vi "SaccadeAnalyser - Main.vi"(8 "error in (no error)":errorcluster, 11 "Data IN":T3={"Impulse Positions"=[{"Start"=5471, "End"=5813, "Impulse Plane"=enum."Yaw", "Impulse Direction +ve?"=FALSE, "Time offset"=0, "Amplitude offset"=0.0}, {"Start"=6974, "End"=7325, "Impulse Plane"=enum."Yaw", "Impulse Direction +ve?"=TRUE, "Time offset"=0, "Amplitude offset"=0.0}, {"Start"=7641, "End"=7980, "Impulse Plane"=enum."Yaw", "Impulse Direction +ve?"=FALSE, "Time offset"=0, "Amplitude offset"=0.0}, {"Start"=9060, "End"=9400, "Impulse Plane"=enum."Yaw", "Impulse Direction +ve?"=FALSE, "Time offset"=0, "Amplitude offset"=0.0}, {"Start"=9938, "End"=10282, "Impulse Plane"=enum."Yaw", "Impulse Direction +ve?"=FALSE, "Time offset"=0, "Amplitude offset"=0.0}, {"Start"=10800, "End"=11142, "Impulse Plane"=enum."Yaw", "Impulse Direction +ve?"=FALSE, "Time offset"=0, "Amplitude offset"=0.0}, {"Start"=11602, "End"=11942, "Impulse Plane"=enum."Yaw", "Impulse Direction +ve?"=TRUE, "Time offset"=0, "Amplitude offset"=0.0}, {"Start"=12449, "End"=12790, "Impulse Plane"=enum."Yaw", "Impulse Direction +ve?"=TRUE, "Time offset"=0, "Amplitude offset"=0.0}, {"Start"=13310, "End"=13653, "Impulse Plane"=enum."Yaw", "Impulse Direction +ve?"=TRUE, "Time offset"=0, "Amplitude offset"=0.0}, {"Start"=14191, "End"=14535, "Impulse Plane"=enum."Yaw", "Impulse Direction +ve?"=TRUE, "Time offset"=0, "Amplitude offset"=0.0}, {"Start"=15040, "End"=15380, "Impulse Plane"=enum."Yaw", "Impulse Direction +ve?"=FALSE, "Time offset"=0, "Amplitude offset"=0.0}, {"Start"=16780, "End"=17124, "Impulse Plane"=enum."Yaw", "Impulse Direction +ve?"=TRUE, "Time offset"=0, "Amplitude offset"=0.0}, {"Start"=17572, "End"=17913, "Impulse Plane"=enum."Yaw", "Impulse Direction +ve?"=FALSE, "Time offset"=0, "Amplitude offset"=0.0}, {"Start"=18369, "End"=18713, "Impulse Plane"=enum."Yaw", "Impulse Direction +ve?"=FALSE, "Time offset"=0, "Amplitude offset"=0.0}, {"Start"=19174, "End"=19519, "Impulse Plane"=enum."Yaw", "Impulse Direction +ve?"=FALSE, "Time offset"=0, "Amplitude offset"=0.0}, {"Start"=19928, "End"=20270, "Impulse Plane"=enum."Yaw", "Impulse Direction +ve?"=TRUE, "Time offset"=0, "Amplitude offset"=0.0}, {"Start"=20762, "End"=21121, "Impulse Plane"=enum."Yaw", "Impulse Direction +ve?"=FALSE, "Time offset"=0, "Amplitude offset"=0.0}, {"Start"=21554, "End"=21888, "Impulse Plane"=enum."Yaw", "Impulse Direction +ve?"=FALSE, "Time offset"=0, "Amplitude offset"=0.0}, {"Start"=22293, "End"=22639, "Impulse Plane"=enum."Yaw", "Impulse Direction +ve?"=TRUE, "Time offset"=0, "Amplitude offset"=0.0}, {"Start"=23109, "End"=23464, "Impulse Plane"=enum."Yaw", "Impulse Direction +ve?"=TRUE, "Time offset"=0, "Amplitude offset"=0.0}, {"Start"=23868, "End"=24215, "Impulse Plane"=enum."Yaw", "Impulse Direction +ve?"=TRUE, "Time offset"=0, "Amplitude offset"=0.0}, {"Start"=24643, "End"=24992, "Impulse Plane"=enum."Yaw", "Impulse Direction +ve?"=FALSE, "Time offset"=0, "Amplitude offset"=0.0}, {"Start"=25685, "End"=26023, "Impulse Plane"=enum."Yaw", "Impulse Direction +ve?"=FALSE, "Time offset"=0, "Amplitude offset"=0.0}, {"Start"=26431, "End"=26768, "Impulse Plane"=enum."Yaw", "Impulse Direction +ve?"=FALSE, "Time offset"=0, "Amplitude offset"=0.0}, {"Start"=27251, "End"=27595, "Impulse Plane"=enum."Yaw", "Impulse Direction +ve?"=FALSE, "Time offset"=0, "Amplitude offset"=0.0}, {"Start"=28832, "End"=29180, "Impulse Plane"=enum."Yaw", "Impulse Direction +ve?"=TRUE, "Time offset"=0, "Amplitude offset"=0.0}, {"Start"=31028, "End"=31383, "Impulse Plane"=enum."LARP", "Impulse Direction +ve?"=FALSE, "Time offset"=0, "Amplitude offset"=0.0}, {"Start"=32603, "End"=32936, "Impulse Plane"=enum."LARP", "Impulse Direction +ve?"=TRUE, "Time offset"=0, "Amplitude offset"=0.0}, {"Start"=33445, "End"=33779, "Impulse Plane"=enum."LARP", "Impulse Direction +ve?"=TRUE, "Time offset"=0, "Amplitude offset"=0.0}, {"Start"=34276, "End"=34629, "Impulse Plane"=enum."LARP", "Impulse Direction +ve?"=FALSE, "Time offset"=0, "Amplitude offset"=0.0}, {"Start"=35114, "End"=35460, "Impulse Plane"=enum."LARP", "Impulse Direction +ve?"=FALSE, "Time offset"=0, "Amplitude offset"=0.0}, {"Start"=35981, "End"=36324, "Impulse Plane"=enum."LARP", "Impulse Direction +ve?"=TRUE, "Time offset"=0, "Amplitude offset"=0.0}, {"Start"=36920, "End"=37249, "Impulse Plane"=enum."LARP", "Impulse Direction +ve?"=TRUE, "Time offset"=0, "Amplitude offset"=0.0}, {"Start"=37988, "End"=38322, "Impulse Plane"=enum."LARP", "Impulse Direction +ve?"=TRUE, "Time offset"=0, "Amplitude offset"=0.0}, {"Start"=38964, "End"=39324, "Impulse Plane"=enum."LARP", "Impulse Direction +ve?"=FALSE, "Time offset"=0, "Amplitude offset"=0.0}, {"Start"=39948, "End"=40284, "Impulse Plane"=enum."LARP", "Impulse Direction +ve?"=TRUE, "Time offset"=0, "Amplitude offset"=0.0}, {"Start"=40958, "End"=41293, "Impulse Plane"=enum."LARP", "Impulse Direction +ve?"=TRUE, "Time offset"=0, "Amplitude offset"=0.0}, {"Start"=41899, "End"=42229, "Impulse Plane"=enum."LARP", "Impulse Direction +ve?"=TRUE, "Time offset"=0, "Amplitude offset"=0.0}, {"Start"=42801, "End"=43154, "Impulse Plane"=enum."LARP", "Impulse Direction +ve?"=FALSE, "Time offset"=0, "Amplitude offset"=0.0}, {"Start"=43641, "End"=43980, "Impulse Plane"=enum."LARP", "Impulse Direction +ve?"=TRUE, "Time offset"=0, "Amplitude offset"=0.0}, {"Start"=44466, "End"=44821, "Impulse Plane"=enum."LARP", "Impulse Direction +ve?"=FALSE, "Time offset"=0, "Amplitude offset"=0.0}, {"Start"=45388, "End"=45722, "Impulse Plane"=enum."LARP", "Impulse Direction +ve?"=TRUE, "Time offset"=0, "Amplitude offset"=0.0}, {"Start"=46149, "End"=46510, "Impulse Plane"=enum."LARP", "Impulse Direction +ve?"=FALSE, "Time offset"=0, "Amplitude offset"=0.0}, {"Start"=47874, "End"=48206, "Impulse Plane"=enum."LARP", "Impulse Direction +ve?"=TRUE, "Time offset"=0, "Amplitude offset"=0.0}, {"Start"=50143, "End"=50479, "Impulse Plane"=enum."RALP", "Impulse Direction +ve?"=TRUE, "Time offset"=0, "Amplitude offset"=0.0}, {"Start"=50976, "End"=51310, "Impulse Plane"=enum."RALP", "Impulse Direction +ve?"=FALSE, "Time offset"=0, "Amplitude offset"=0.0}, {"Start"=51892, "End"=52226, "Impulse Plane"=enum."RALP", "Impulse Direction +ve?"=FALSE, "Time offset"=0, "Amplitude offset"=0.0}, {"Start"=52839, "End"=53171, "Impulse Plane"=enum."RALP", "Impulse Direction +ve?"=FALSE, "Time offset"=0, "Amplitude offset"=0.0}, {"Start"=53676, "End"=54012, "Impulse Plane"=enum."RALP", "Impulse Direction +ve?"=TRUE, "Time offset"=0, "Amplitude offset"=0.0}, {"Start"=54530, "End"=54877, "Impulse Plane"=enum."RALP", "Impulse Direction +ve?"=FALSE, "Time offset"=0, "Amplitude offset"=0.0}, {"Start"=55371, "End"=55711, "Impulse Plane"=enum."RALP", "Impulse Direction +ve?"=TRUE, "Time offset"=0, "Amplitude offset"=0.0}, {"Start"=56153, "End"=56482, "Impulse Plane"=enum."RALP", "Impulse Direction +ve?"=FALSE, "Time offset"=0, "Amplitude offset"=0.0}, {"Start"=57053, "End"=57390, "Impulse Plane"=enum."RALP", "Impulse Direction +ve?"=FALSE, "Time offset"=0, "Amplitude offset"=0.0}, {"Start"=57954, "End"=58292, "Impulse Plane"=enum."RALP", "Impulse Direction +ve?"=FALSE, "Time offset"=0, "Amplitude offset"=0.0}, {"Start"=58794, "End"=59130, "Impulse Plane"=enum."RALP", "Impulse Direction +ve?"=TRUE, "Time offset"=0, "Amplitude offset"=0.0}, {"Start"=59587, "End"=59931, "Impulse Plane"=enum."RALP", "Impulse Direction +ve?"=TRUE, "Time offset"=0, "Amplitude offset"=0.0}, {"Start"=60399, "End"=60744, "Impulse Plane"=enum."RALP", "Impulse Direction +ve?"=FALSE, "Time offset"=0, "Amplitude offset"=0.0}, {"Start"=61218, "End"=61559, "Impulse Plane"=enum."RALP", "Impulse Direction +ve?"=FALSE, "Time offset"=0, "Amplitude offset"=0.0}, {"Start"=62100, "End"=62442, "Impulse Plane"=enum."RALP", "Impulse Direction +ve?"=FALSE, "Time offset"=0, "Amplitude offset"=0.0}, {"Start"=62989, "End"=63322, "Impulse Plane"=enum."RALP", "Impulse Direction +ve?"=FALSE, "Time offset"=0, "Amplitude offset"=0.0}, {"Start"=63787, "End"=64136, "Impulse Plane"=enum."RALP", "Impulse Direction +ve?"=TRUE, "Time offset"=0, "Amplitude offset"=0.0}, {"Start"=64603, "End"=64953, "Impulse Plane"=enum."RALP", "Impulse Direction +ve?"=FALSE, "Time offset"=0, "Amplitude offset"=0.0}, {"Start"=65462, "End"=65795, "Impulse Plane"=enum."RALP", "Impulse Direction +ve?"=FALSE, "Time offset"=0, "Amplitude offset"=0.0}, {"Start"=66308, "End"=66645, "Impulse Plane"=enum."RALP", "Impulse Direction +ve?"=FALSE, "Time offset"=0, "Amplitude offset"=0.0}, {"Start"=67052, "End"=67402, "Impulse Plane"=enum."RALP", "Impulse Direction +ve?"=TRUE, "Time offset"=0, "Amplitude offset"=0.0}], "No. Imp"=15, "Parameter Time Series"=[{"time offset"=0.0, "Offset"=0.0, "Gain"=1.0, "inverse"=FALSE, "filter data"=FALSE, "dots"=FALSE, "interpolate"=FALSE, "List 1"=5, "Color Box"=6618880, "Boolean"=TRUE}, {"time offset"=0.0, "Offset"=0.0, "Gain"=1.0, "inverse"=FALSE, "filter data"=FALSE, "dots"=FALSE, "interpolate"=FALSE, "List 1"=6, "Color Box"=6618880, "Boolean"=FALSE}, {"time offset"=0.0, "Offset"=0.0, "Gain"=1.0, "inverse"=FALSE, "filter data"=FALSE, "dots"=FALSE, "interpolate"=FALSE, "List 1"=7, "Color Box"=6618880, "Boolean"=FALSE}, {"time offset"=0.0, "Offset"=0.0, "Gain"=1.0, "inverse"=FALSE, "filter data"=FALSE, "dots"=FALSE, "interpolate"=FALSE, "List 1"=13, "Color Box"=16777224, "Boolean"=TRUE}, {"time offset"=0.0, "Offset"=0.0, "Gain"=1.0, "inverse"=FALSE, "filter data"=FALSE, "dots"=FALSE, "interpolate"=FALSE, "List 1"=14, "Color Box"=16777224, "Boolean"=FALSE}, {"time offset"=0.0, "Offset"=0.0, "Gain"=1.0, "inverse"=FALSE, "filter data"=FALSE, "dots"=FALSE, "interpolate"=FALSE, "List 1"=15, "Color Box"=16777224, "Boolean"=FALSE}], "Parameter Impuls Series"=[{"Color"=6618880, "Visible"=TRUE, "Channel"=1, "Invert"=FALSE, "Desaccade"=FALSE, "Offset"=0.0, "Gain"=1.0}, {"Color"=6618880, "Visible"=FALSE, "Channel"=6, "Invert"=FALSE, "Desaccade"=FALSE, "Offset"=0.0, "Gain"=1.0}, {"Color"=6618880, "Visible"=FALSE, "Channel"=7, "Invert"=FALSE, "Desaccade"=FALSE, "Offset"=0.0, "Gain"=1.0}, {"Color"=16777224, "Visible"=TRUE, "Channel"=13, "Invert"=FALSE, "Desaccade"=FALSE, "Offset"=0.0, "Gain"=1.0}, {"Color"=16777224, "Visible"=FALSE, "Channel"=14, "Invert"=FALSE, "Desaccade"=FALSE, "Offset"=0.0, "Gain"=1.0}, {"Color"=16777224, "Visible"=FALSE, "Channel"=15, "Invert"=FALSE, "Desaccade"=FALSE, "Offset"=0.0, "Gain"=1.0}], "Experiment Parameters"={"Freq"=0.0, "Vel"=0, "Acc"=0, "Stimulus"="Head Impulse"}, "Autosort File"=refnum, "Data File"={"Data Channels"=array34x71049[2415666 elements], "Sample Rate"=500, "Channel List"=["Hz Position-in-Head", "Hz Velocity-in-Head", "Hy Position-in-Head", "Hy Velocity-in-Head", "Hx Position-in-Head", "Hx Velocity-in-Head", "Hl Velocity-in-Head", "Hr Velocity-in-Head", "Lx Position-in-Head", "Ly Position-in-Head", "Lz Position-in-Head", "Lx Velocity-in-Head", "Ly Velocity-in-Head", "Lz Velocity-in-Head", "Ll Velocity-in-Head", "Lr Velocity-in-Head", "Rx Position-in-Head", "Ry Position-in-Head", "Rz Position-in-Head", "Rx Velocity-in-Head", "Ry Velocity-in-Head", "Rz Velocity-in-Head", "Rl Velocity-in-Head", "Rr Velocity-in-Head", "Target on/off", "aux input 1", "aux input 2", " ", "", "", "", "Target Hor", "Target Ver", ""]}, "Experiment data path"=path "C:/Users/w.figtree/Desktop/Coils Data/3", "Image data path"=path "/Macintosh HD/Users/patrick/Studium/Diploma Thesis/Data Analysis", "LVS data path"=path "/Macintosh HD/Users/patrick/Studium/Diploma Thesis/Data Analysis", "Raw copy path"=path "/Macintosh HD/Users/patrick/Studium/Diploma Thesis/Data Analysis", "filename"="passive_lvs.lvs", "desaccading parameters"={"Tolerance"=3, "Acc Range"=7000.0, "Sample Rate"=500, "Impulse Plane 2"=enum."Yaw", "Impulse dir"=FALSE}, "Experiment Parameters 2"={"Subject"="SE Trial Short Term", "Strain"="", "Rotation plane"="", "Experimenter"=" ", "Trial"=0.0, "Time"=0.0}, "Excel"={"Excel._Application"=refnum, "Use Excel"=TRUE, "Worksheet SINE"=refnum, "Row SINE"=0, "Worksheet TRANS"=refnum, "Row TRANS"=0}, "Session Config File"=refnum, "Autosort Parameter Set"=4, "EMA Version"="EMA 2016a", "desacc "={"Threshold 1 [Acc]"=7000.0, "Threshold 2 [% of TH1]"=60, "tolerance"=3, "Search WD "=0.1, " always use TH2"=FALSE, "Range"=3.0, "Max time"=120.0, "Min time"=20.0, "Velocity Threshold"=150}, "Cycle Nr for Saccades"={"POS"=0, "NEG"=0}, "calibration name"="u_calibration_1_p00001s001_calib.mat", "Excel"=refnum} {"Parameter Time Series"."time offset" format="%.3f"; "Parameter Time Series"."Gain" format="%.1f"; "Parameter Time Series"."Offset" format="%.1f"; "Parameter Time Series"."List 1" items=["Motor-Pos", "Motor-Vel", "Lx Position-in-Head", "Ly Position-in-Head", "Lz Position-in-Head", "Lx Velocity-in-Head", "Ly Velocity-in-Head", "Lz Velocity-in-Head", "Ll Velocity-in-Head", "Lr Velocity-in-Head", "Lx Accel-in-Head", "Ly Accel-in-Head", "Lz Accel-in-Head", "Rx Position-in-Head", "Ry Position-in-Head", "Rz Position-in-Head", "Rx Velocity-in-Head", "Ry Velocity-in-Head", "Rz Velocity-in-Head", "Rl Velocity-in-Head", "Rr Velocity-in-Head", "Rx Accel-in-Head", "Ry Accel-in-Head", "Rz Accel-in-Head", "Global Trigger", "", "", ""]; "Parameter Impuls Series"."Gain" format="%.1f"; "Parameter Impuls Series"."Offset" format="%.1f"}) -> (0 "error out":errorcluster, 3 "Data OUT":T3={"Impulse Positions"=[{"Start"=5471, "End"=5813, "Impulse Plane"=enum."Yaw", "Impulse Direction +ve?"=FALSE, "Time offset"=0, "Amplitude offset"=0.0}, {"Start"=6974, "End"=7325, "Impulse Plane"=enum."Yaw", "Impulse Direction +ve?"=TRUE, "Time offset"=0, "Amplitude offset"=0.0}, {"Start"=7641, "End"=7980, "Impulse Plane"=enum."Yaw", "Impulse Direction +ve?"=FALSE, "Time offset"=0, "Amplitude offset"=0.0}, {"Start"=9060, "End"=9400, "Impulse Plane"=enum."Yaw", "Impulse Direction +ve?"=FALSE, "Time offset"=0, "Amplitude offset"=0.0}, {"Start"=9938, "End"=10282, "Impulse Plane"=enum."Yaw", "Impulse Direction +ve?"=FALSE, "Time offset"=0, "Amplitude offset"=0.0}, {"Start"=10800, "End"=11142, "Impulse Plane"=enum."Yaw", "Impulse Direction +ve?"=FALSE, "Time offset"=0, "Amplitude offset"=0.0}, {"Start"=11602, "End"=11942, "Impulse Plane"=enum."Yaw", "Impulse Direction +ve?"=TRUE, "Time offset"=0, "Amplitude offset"=0.0}, {"Start"=12449, "End"=12790, "Impulse Plane"=enum."Yaw", "Impulse Direction +ve?"=TRUE, "Time offset"=0, "Amplitude offset"=0.0}, {"Start"=13310, "End"=13653, "Impulse Plane"=enum."Yaw", "Impulse Direction +ve?"=TRUE, "Time offset"=0, "Amplitude offset"=0.0}, {"Start"=14191, "End"=14535, "Impulse Plane"=enum."Yaw", "Impulse Direction +ve?"=TRUE, "Time offset"=0, "Amplitude offset"=0.0}, {"Start"=15040, "End"=15380, "Impulse Plane"=enum."Yaw", "Impulse Direction +ve?"=FALSE, "Time offset"=0, "Amplitude offset"=0.0}, {"Start"=16780, "End"=17124, "Impulse Plane"=enum."Yaw", "Impulse Direction +ve?"=TRUE, "Time offset"=0, "Amplitude offset"=0.0}, {"Start"=17572, "End"=17913, "Impulse Plane"=enum."Yaw", "Impulse Direction +ve?"=FALSE, "Time offset"=0, "Amplitude offset"=0.0}, {"Start"=18369, "End"=18713, "Impulse Plane"=enum."Yaw", "Impulse Direction +ve?"=FALSE, "Time offset"=0, "Amplitude offset"=0.0}, {"Start"=19174, "End"=19519, "Impulse Plane"=enum."Yaw", "Impulse Direction +ve?"=FALSE, "Time offset"=0, "Amplitude offset"=0.0}, {"Start"=19928, "End"=20270, "Impulse Plane"=enum."Yaw", "Impulse Direction +ve?"=TRUE, "Time offset"=0, "Amplitude offset"=0.0}, {"Start"=20762, "End"=21121, "Impulse Plane"=enum."Yaw", "Impulse Direction +ve?"=FALSE, "Time offset"=0, "Amplitude offset"=0.0}, {"Start"=21554, "End"=21888, "Impulse Plane"=enum."Yaw", "Impulse Direction +ve?"=FALSE, "Time offset"=0, "Amplitude offset"=0.0}, {"Start"=22293, "End"=22639, "Impulse Plane"=enum."Yaw", "Impulse Direction +ve?"=TRUE, "Time offset"=0, "Amplitude offset"=0.0}, {"Start"=23109, "End"=23464, "Impulse Plane"=enum."Yaw", "Impulse Direction +ve?"=TRUE, "Time offset"=0, "Amplitude offset"=0.0}, {"Start"=23868, "End"=24215, "Impulse Plane"=enum."Yaw", "Impulse Direction +ve?"=TRUE, "Time offset"=0, "Amplitude offset"=0.0}, {"Start"=24643, "End"=24992, "Impulse Plane"=enum."Yaw", "Impulse Direction +ve?"=FALSE, "Time offset"=0, "Amplitude offset"=0.0}, {"Start"=25685, "End"=26023, "Impulse Plane"=enum."Yaw", "Impulse Direction +ve?"=FALSE, "Time offset"=0, "Amplitude offset"=0.0}, {"Start"=26431, "End"=26768, "Impulse Plane"=enum."Yaw", "Impulse Direction +ve?"=FALSE, "Time offset"=0, "Amplitude offset"=0.0}, {"Start"=27251, "End"=27595, "Impulse Plane"=enum."Yaw", "Impulse Direction +ve?"=FALSE, "Time offset"=0, "Amplitude offset"=0.0}, {"Start"=28832, "End"=29180, "Impulse Plane"=enum."Yaw", "Impulse Direction +ve?"=TRUE, "Time offset"=0, "Amplitude offset"=0.0}, {"Start"=31028, "End"=31383, "Impulse Plane"=enum."LARP", "Impulse Direction +ve?"=FALSE, "Time offset"=0, "Amplitude offset"=0.0}, {"Start"=32603, "End"=32936, "Impulse Plane"=enum."LARP", "Impulse Direction +ve?"=TRUE, "Time offset"=0, "Amplitude offset"=0.0}, {"Start"=33445, "End"=33779, "Impulse Plane"=enum."LARP", "Impulse Direction +ve?"=TRUE, "Time offset"=0, "Amplitude offset"=0.0}, {"Start"=34276, "End"=34629, "Impulse Plane"=enum."LARP", "Impulse Direction +ve?"=FALSE, "Time offset"=0, "Amplitude offset"=0.0}, {"Start"=35114, "End"=35460, "Impulse Plane"=enum."LARP", "Impulse Direction +ve?"=FALSE, "Time offset"=0, "Amplitude offset"=0.0}, {"Start"=35981, "End"=36324, "Impulse Plane"=enum."LARP", "Impulse Direction +ve?"=TRUE, "Time offset"=0, "Amplitude offset"=0.0}, {"Start"=36920, "End"=37249, "Impulse Plane"=enum."LARP", "Impulse Direction +ve?"=TRUE, "Time offset"=0, "Amplitude offset"=0.0}, {"Start"=37988, "End"=38322, "Impulse Plane"=enum."LARP", "Impulse Direction +ve?"=TRUE, "Time offset"=0, "Amplitude offset"=0.0}, {"Start"=38964, "End"=39324, "Impulse Plane"=enum."LARP", "Impulse Direction +ve?"=FALSE, "Time offset"=0, "Amplitude offset"=0.0}, {"Start"=39948, "End"=40284, "Impulse Plane"=enum."LARP", "Impulse Direction +ve?"=TRUE, "Time offset"=0, "Amplitude offset"=0.0}, {"Start"=40958, "End"=41293, "Impulse Plane"=enum."LARP", "Impulse Direction +ve?"=TRUE, "Time offset"=0, "Amplitude offset"=0.0}, {"Start"=41899, "End"=42229, "Impulse Plane"=enum."LARP", "Impulse Direction +ve?"=TRUE, "Time offset"=0, "Amplitude offset"=0.0}, {"Start"=42801, "End"=43154, "Impulse Plane"=enum."LARP", "Impulse Direction +ve?"=FALSE, "Time offset"=0, "Amplitude offset"=0.0}, {"Start"=43641, "End"=43980, "Impulse Plane"=enum."LARP", "Impulse Direction +ve?"=TRUE, "Time offset"=0, "Amplitude offset"=0.0}, {"Start"=44466, "End"=44821, "Impulse Plane"=enum."LARP", "Impulse Direction +ve?"=FALSE, "Time offset"=0, "Amplitude offset"=0.0}, {"Start"=45388, "End"=45722, "Impulse Plane"=enum."LARP", "Impulse Direction +ve?"=TRUE, "Time offset"=0, "Amplitude offset"=0.0}, {"Start"=46149, "End"=46510, "Impulse Plane"=enum."LARP", "Impulse Direction +ve?"=FALSE, "Time offset"=0, "Amplitude offset"=0.0}, {"Start"=47874, "End"=48206, "Impulse Plane"=enum."LARP", "Impulse Direction +ve?"=TRUE, "Time offset"=0, "Amplitude offset"=0.0}, {"Start"=50143, "End"=50479, "Impulse Plane"=enum."RALP", "Impulse Direction +ve?"=TRUE, "Time offset"=0, "Amplitude offset"=0.0}, {"Start"=50976, "End"=51310, "Impulse Plane"=enum."RALP", "Impulse Direction +ve?"=FALSE, "Time offset"=0, "Amplitude offset"=0.0}, {"Start"=51892, "End"=52226, "Impulse Plane"=enum."RALP", "Impulse Direction +ve?"=FALSE, "Time offset"=0, "Amplitude offset"=0.0}, {"Start"=52839, "End"=53171, "Impulse Plane"=enum."RALP", "Impulse Direction +ve?"=FALSE, "Time offset"=0, "Amplitude offset"=0.0}, {"Start"=53676, "End"=54012, "Impulse Plane"=enum."RALP", "Impulse Direction +ve?"=TRUE, "Time offset"=0, "Amplitude offset"=0.0}, {"Start"=54530, "End"=54877, "Impulse Plane"=enum."RALP", "Impulse Direction +ve?"=FALSE, "Time offset"=0, "Amplitude offset"=0.0}, {"Start"=55371, "End"=55711, "Impulse Plane"=enum."RALP", "Impulse Direction +ve?"=TRUE, "Time offset"=0, "Amplitude offset"=0.0}, {"Start" (continued)
-95.17389475330742, -86.42835772109143, -77.50279294410363, -68.49624407599312, -59.51012539199722, -50.64704208212082, -41.987514476015996, -33.57432674148718, -25.423987627866047, -17.53729863914719, -9.910820909812287, -2.5483350434714613, 4.535845876246067, 11.308975939205853, 17.718236979256062, 23.696731611338603, 29.177332668897733, 34.10513667258561, 38.440614925997224, 42.160594620075706, 45.260369681709, 47.75135796127779, 49.65226955051388, 50.9906360208702, 51.79800888798371, 52.107702902138215, 51.96045824284653, 51.395202055156055, 50.45297325544797, 49.18285273665435, 47.629439626256385, 45.828514343973026, 43.813895445590475, 41.61597526624965, 39.2613760407162, 36.78004246010816, 34.19988033209459, 31.554138919269807, 28.8840016476756, 26.22160520523843, 23.59096490914682, 21.01509885239349, 18.511543541868093, 16.086055171893662, 13.749669048039907, 11.52687305953824, 9.442591317601064, 7.522911882619418, 5.786741415409173, 4.235773882363097, 2.8527140148095196, 1.602268357345808, 0.4347609925677234, -0.6992749780891954, -1.8254185814913066, -2.9525609863646674, -4.073613136931928, -5.14819166339495, -6.121013743080621, -6.9438443591398595, -7.580544193359222, -8.016057622746764, -8.251523577558732, -8.296487862562273, -8.16986736892337, -7.898051795121088, -7.502048365612218, -6.985750347252864, -6.35132857331239, -5.615455540123179, -4.799893545694648, -3.9299394950044366, -3.047680064582874, -2.200607298897424, -1.4271571748228133, -0.750068695431203, -0.16334991046952752, 0.36075943030685664, 0.8643327530523806, 1.403460879250897, 2.030328712078621, 2.7743416245535357, 3.634780782393193, 4.577021368037045, 5.542736921808352, 6.462650598144727, 7.258845262864778, 7.866378999330756, 8.248955120243387, 8.395952645738607, 8.32878021705643, 8.098213070404832, 7.770817101514378, 7.417043453176731, 7.102829375465877, 6.878414380003594, 6.767337835570437, 6.769116698443309, 6.862636131561903, 7.008097751570517, 7.153932533487, 7.247260267321646, 7.237985508007169, 7.085512613613966, 6.7785498563182855, 6.330561431456207, 5.771025689887551, 5.155802872961214, 4.5573597144135904, 4.044910224031232, 3.6718031904539803, 3.461163107296736, 3.400847628687603, 3.4497326836835516, 3.541718228167298, 3.5917837927962197, 3.5206566080189976, 3.281140063293118, 2.861985911357511, 2.286552098924709, 1.61524339750927, 0.9356137751130742, 0.3388576693563894, -0.0995874318773784, -0.338178197026092, -0.3763014212648714, -0.24540391273728956, -0.005972186540577518, 0.2599752413497929, 0.4697935173424064, 0.5671637390756716, 0.5323829854142619, 0.37551523398971165, 0.13099858887954996, -0.14748123514985068, -0.39789876110009126, -0.5692899842141106, -0.6355660883685377, -0.5983427889259292, -0.4857862859002826, -0.3447652979593576, -0.22655901420659408, -0.17042292361397005, -0.18290222263566447, -0.23011006163415404, -0.24844682022715858, -0.15841153045381495, 0.11397290720116948, 0.6119602967729127, 1.325717080521212, 2.1846708899897007, 3.0701028609386, 3.833907555939943, 4.332113921068256, 4.465830512513329, 4.207369847178844, 3.6096178154160126, 2.793870629607797, 1.9243170305465243, 1.1756320919365963, 0.6909788478892734, 0.5511144364034996, 0.7654991213032871, 1.2791044240513083, 1.9868451397526505, 2.7615426719135323, 3.4883261049675496, 4.079362556260325, 4.482772178377651, 4.684915419412732, 4.705671814749792, 4.592361102477108, 4.400029317630196, 4.173840645363373, 3.9487501596973864, 3.754964931001955, 3.6123670828772183, 3.5255531273093483, 3.4914329064213274, 3.5021944296200167, 3.545841693841248, 3.612572706665807, 3.6888657363279114, 3.7625250816761033, 3.836402868947848, 3.9206231234724216, 4.02532304449381, 4.166115543466246, 4.36103739310933, 4.617644939374388, 4.933441599220007, 5.291941564563578, 5.660259851836125, 6.004533273598341, 6.296355287206681]}, {[0.0, 2.0, 4.0, 6.0, 8.0, 10.0, 12.0, 14.0, 16.0, 18.000000000000004, 20.0, 22.0, 24.0, 26.000000000000004, 28.0, 30.0, 32.0, 34.0, 36.00000000000001, 38.0, 40.0, 42.0, 44.0, 46.0, 48.0, 50.0, 52.00000000000001, 54.0, 56.0, 58.0, 60.0, 62.0, 64.0, 66.0, 68.0, 70.0, 72.00000000000001, 74.0, 76.0, 78.0, 80.0, 82.0, 84.0, 86.0, 88.0, 90.0, 92.0, 94.0, 96.0, 98.0, 100.0, 102.00000000000001, 104.00000000000001, 106.0, 108.0, 110.0, 112.0, 114.0, 116.0, 118.00000000000001, 120.0, 122.0, 124.0, 126.0, 128.0, 130.0, 132.0, 134.0, 136.0, 138.0, 140.0, 142.00000000000003, 144.00000000000003, 146.0, 148.0, 150.0, 152.0, 154.0, 156.0, 158.0, 160.0, 162.0, 164.0, 166.0, 168.0, 170.0, 172.0, 174.00000000000003, 176.0, 178.0, 180.0, 182.0, 184.0, 186.0, 188.0, 190.0, 192.0, 194.0, 196.0, 198.0, 200.0, 202.0, 204.00000000000003, 206.00000000000003, 208.00000000000003, 210.0, 212.0, 214.0, 216.0, 218.0, 220.0, 222.0, 224.0, 226.0, 228.0, 230.0, 232.0, 234.0, 236.00000000000003, 238.00000000000003, 240.0, 242.0, 244.0, 246.0, 248.0, 250.0, 252.0, 254.0, 256.0, 258.0, 260.0, 262.0, 264.0, 266.0, 268.0, 270.0, 272.0, 274.0, 276.0, 278.0, 280.0, 282.0, 284.00000000000006, 286.00000000000006, 288.00000000000006, 290.0, 292.0, 294.0, 296.0, 298.0, 300.0, 302.0, 304.0, 306.0, 308.0, 310.0, 312.0, 314.0, 316.0, 318.0, 320.0, 322.0, 324.0, 326.0, 328.0, 330.0, 332.0, 334.0, 336.0, 338.0, 340.0, 342.0, 344.0, 346.00000000000006, 348.00000000000006, 350.00000000000006, 352.0, 354.0, 356.0, 358.0, 360.0, 362.0, 364.0, 366.0, 368.0, 370.0, 372.0, 374.0, 376.0, 378.0, 380.0, 382.0, 384.0, 386.0, 388.0, 390.0, 392.0, 394.0, 396.0, 398.0, 400.0, 402.0, 404.0, 406.0, 408.00000000000006, 410.00000000000006, 412.00000000000006, 414.00000000000006, 416.00000000000006, 418.0, 420.0, 422.0, 424.0, 426.0, 428.0, 430.0, 432.0, 434.0, 436.0, 438.0, 440.0, 442.0, 444.0, 446.0, 448.0, 450.0, 452.0, 454.0, 456.0, 458.0, 460.0, 462.0, 464.0, 466.0, 468.0, 470.00000000000006, 472.00000000000006, 474.00000000000006, 476.00000000000006, 478.00000000000006, 480.0, 482.0, 484.0, 486.0, 488.0, 490.0, 492.0, 494.0, 496.0, 498.0, 500.0, 502.0, 504.0, 506.0, 508.0, 510.0, 512.0, 514.0, 516.0, 518.0, 520.0, 522.0, 524.0, 526.0, 528.0, 530.0, 532.0, 534.0, 536.0, 538.0, 540.0, 542.0, 544.0, 546.0, 548.0, 550.0, 552.0, 554.0, 556.0, 558.0, 560.0, 562.0, 564.0, 566.0000000000001, 568.0000000000001, 570.0000000000001, 572.0000000000001, 574.0000000000001, 576.0000000000001, 578.0, 580.0, 582.0, 584.0, 586.0, 588.0, 590.0, 592.0, 594.0, 596.0, 598.0, 600.0, 602.0, 604.0, 606.0, 608.0, 610.0, 612.0, 614.0, 616.0, 618.0, 620.0, 622.0, 624.0, 626.0, 628.0, 630.0, 632.0, 634.0, 636.0, 638.0, 640.0, 642.0, 644.0, 646.0, 648.0, 650.0, 652.0, 654.0, 656.0, 658.0, 660.0, 662.0, 664.0, 666.0, 668.0], [0.265610379123574, 0.29955438385781186, 0.3073271510825837, 0.25088170996927195, 0.0955778657182802, -0.17967780777815423, -0.5751722734804205, -1.0677018531375335, -1.61100903009555, -2.1376998735894435, -2.572438221453584, -2.845032069711387, -2.889990796852881, -2.6640254261804124, -2.1589385237368877, -1.3973704532581044, -0.4410262669261744, 0.6149625202148918, 1.6578105645927366, 2.568811085746651, 3.2405719488554574, 3.594418236019102, 3.59423134311362, 3.25426604455523, 2.638589170647734, 1.8522212693232056, 1.024002842924581, 0.28363083535791134, -0.2631273413804074, -0.5479879756193711, -0.5526599718088967, -0.3165667427949188, 0.08194754174687802, 0.5427040166793802, 0.9601126465967837, 1.2490660941795717, 1.3552494917380287, 1.2609660266111007, 0.9901061006760159, 0.5929500171323312, 0.1316452102061163, -0.3242014734115539, -0.7070448072580895, -0.9576555053270059, -1.0308656102396565, -0.9028966409212558, -0.5706475885558007, -0.05640306293182107, 0.5878774319182494, 1.2919795402292316, 1.9752603217813292, 2.544460261904801, 2.9108640058497013, 3.02292719395402, 2.8769591618105945, 2.5096872837018456, 1.9994145171867412, 1.4589149733005922, 1.0130301435033422, 0.779086879194411, 0.8388205094944912, 1.2193460895300507, 1.8972037136660749, 2.7947866523875557, 3.7991173162436107, 4.79963073632729, 5.706612873787008, 6.471272891430737, 7.098232848455165, 7.6399749071079235, 8.182260651278948, 8.816664249741773, 9.608676400714568, 10.581690618744048, 11.714448887827388, 12.944304963363857, 14.181649380388317, 15.341814236572201, 16.36898520101776, 17.251037369821923, 18.02771079795455, 18.774737655569943, 19.59660607980983, 20.609548279379887, 21.910493852368674, 23.564991322059484, 25.599038915860945, 27.995354138312287, 30.698245013489952, 33.621538845141956, 36.660697549428775, 39.71088248492803, 42.68703386391552, 45.54350379296848, 48.27638299599656, 50.92001657734758, 53.551649661511235, 56.28460062906045, 59.23880951581975, 62.509165157283164, 66.15706942297979, 70.1813388433286, 74.50222978959407, 78.9920946850517, 83.49515768393319, 87.85398915379608, 91.95720661922029, 95.76601760083558, 99.31875528542986, 102.732062215853, 106.17671834454964, 109.83013317991686, 113.83681511996252, 118.27414113622005, 123.13105350414074, 128.31320726079903, 133.6641703987848, 138.99545910078118, 144.1223586303302, 148.89579947533664, 153.22971027773622, 157.11441168936207, 160.60993560225924, 163.8360106182837, 166.94977164161065, 170.11109167488672, 173.4496844604976, 177.0325311095539, 180.8358671832565, 184.7434535685395, 188.55846961042656, 192.0302120782026, 194.91361150677585, 197.02462915597096, 198.27654675071486, 198.70441047367206, 198.465230865703, 197.79568521254288, 196.94452323551602, 196.1076320934, 195.3715139051856, 194.68128329964304, 193.85426001254115, 192.63098444427644, 190.73203379501064, 187.92977958785724, 184.11421329468334, 179.32036958585968, 173.71665747967893, 167.55375366090098, 161.11118007895197, 154.6360289998317, 148.28666184003117, 142.11754781311117, 136.08844273826375, 130.1048549647473, 124.06617982459825, 117.89503276002162, 111.56058155119892, 105.08344915768772, 98.52216713045169, 91.93980994679826, 85.37460261371703, 78.83762245568018, 72.31597805612617, 65.78261955393609, 59.21217422677118, 52.60364667870252, 45.99332845065388, 39.4495543624806, 33.06759489362736, 26.94745149891321, 21.168779987935444, 15.789543553990821, 10.841424500395116, 6.329389831814105, 2.243338406300916, -1.4408024113097442, -4.753198611115494, -7.715157342228786, -10.349980679517849, -12.685283947905305, -14.74347678518214, -16.54672988568731, -18.119532592223184, -19.492800757323025, -20.69050763673577, -21.731545803107586, -22.644341132823428, -23.45514838089197, -24.181695187699802, -24.83795046912732, -25.424081666155807, -25.91671622426051, -26.28054167758647, -26.46408127824203, -26.41006487056076, -26.08885858570484, -25.498978933335163, -24.671599665560596, -23.681234846942544, -22.625611141220148, -21.60835656475544, -20.725592921982013, -20.033919556493956, -19.53325705408497, -19.1835239405942, -18.918407332943953, -18.651778862235552, -18.299287489711574, -17.80598565425531, -17.160013747803468, -16.381532408590893, -15.513713246272543, -14.609932782284748, -13.711801871896416, -12.853869639116839, -12.063364564929222, -11.355392193105018, -10.743861349029878, -10.233895770866923, -9.825336952579892, -9.528703382656975, -9.344803696431146, -9.257859405380085, -9.248670081700443, -9.292211526962074, -9.362232844666242, -9.440999937828689, -9.523339050315375, -9.62162825642581, -9.76484402592709, -9.988248346718795, -10.319267984034436, -10.76882045505652, -11.32809453440618, -11.954173677051799, -12.573633982598949, -13.104848059626043, -13.475154407481737, -13.63351721134833, -13.567934642071979, -13.31548193192049, -12.948115550068117, -12.555870666454037, -12.21526187981424, -11.960323181384728, -11.78734516550761, -11.647081754674058, -11.447577167297608, -11.096914094001088, -10.536415299443867, -9.772855209759085, -8.905697006175616, -8.115386023058287, -7.625369066130714, -7.658105027938794, -8.360802550755661, -9.709972315585073, -11.4476193776905, -13.068851678881895, -13.862730914838576, -12.99963998702583, -9.694639981902103, -3.402083180014002, 6.032556885524558, 18.251678113366445, 32.3514578152284, 46.96196273804698, 60.41458212174757, 71.01485846520777, 77.33772940656948, 78.468047531521, 74.18538908447246, 65.01631412660365, 52.128564083566516, 37.14123702954777, 21.855399138477154, 7.934316510732438, -3.3578249787371295, -11.309186108976784, -15.805578117508423, -17.26506975033719, -16.46631522978143, -14.335344694369246, -11.750138041033814, -9.391172054249932, -7.662753402156021, -6.689280610156021, -6.37899976114219, -6.512846891324843, -6.839819227844784, -7.16165158164653, -7.361303101770953, -7.39529221470326, -7.282769964902262, -7.071567134844985, -6.811430703794715, -6.549679759979784, -6.316784366634206, -6.128991166364515, -6.001872665363912, -5.956241747729779, -6.014021184265944, -6.183619648149296, -6.444300716355462, -6.752798948024768, -7.063490238626905, -7.323653484500898, -7.488171882105775, -7.544345032809517, -7.511730789578261, -7.424989355798693, -7.324146499725459, -7.253553191908345, -7.228762672612359, -7.226601965262125, -7.206410650471126, -7.122081119060683, -6.9522298225814465, -6.719792570120703, -6.484379371887826, -6.336725379856866, -6.374763841912424, -6.664152474176003, -7.214056936778066, -7.966216797721388, -8.801977403007834, -9.57128359722487, -10.14182957413143, -10.432953065009226, -10.437026858052217, -10.234727810726625, -9.963996049045846]}, {[0.0, 2.0, 4.0, 6.0, 8.0, 10.0, 12.0, 14.0, 16.0, 18.000000000000004, 20.0, 22.0, 24.0, 26.000000000000004, 28.0, 30.0, 32.0, 34.0, 36.00000000000001, 38.0, 40.0, 42.0, 44.0, 46.0, 48.0, 50.0, 52.00000000000001, 54.0, 56.0, 58.0, 60.0, 62.0, 64.0, 66.0, 68.0, 70.0, 72.00000000000001, 74.0, 76.0, 78.0, 80.0, 82.0, 84.0, 86.0, 88.0, 90.0, 92.0, 94.0, 96.0, 98.0, 100.0, 102.00000000000001, 104.00000000000001, 106.0, 108.0, 110.0, 112.0, 114.0, 116.0, 118.00000000000001, 120.0, 122.0, 124.0, 126.0, 128.0, 130.0, 132.0, 134.0, 136.0, 138.0, 140.0, 142.00000000000003, 144.00000000000003, 146.0, 148.0, 150.0, 152.0, 154.0, 156.0, 158.0, 160.0, 162.0, 164.0, 166.0, 168.0, 170.0, 172.0, 174.00000000000003, 176.0, 178.0, 180.0, 182.0, 184.0, 186.0, 188.0, 190.0, 192.0, 194.0, 196.0, 198.0, 200.0, 202.0, 204.00000000000003, 206.00000000000003, 208.00000000000003, 210.0, 212.0, 214.0, 216.0, 218.0, 220.0, 222.0, 224.0, 226.0, 228.0, 230.0, 232.0, 234.0, 236.00000000000003, 238.00000000000003, 240.0, 242.0, 244.0, 246.0, 248.0, 250.0, 252.0, 254.0, 256.0, 258.0, 260.0, 262.0, 264.0, 266.0, 268.0, 270.0, 272.0, 274.0, 276.0, 278.0, 280.0, 282.0, 284.00000000000006, 286.00000000000006, 288.00000000000006, 290.0, 292.0, 294.0, 296.0, 298.0, 300.0, 302.0, 304.0, 306.0, 308.0, 310.0, 312.0, 314.0, 316.0, 318.0, 320.0, 322.0, 324.0, 326.0, 328.0, 330.0, 332.0, 334.0, 336.0, 338.0, 340.0, 342.0, 344.0, 346.00000000000006, 348.00000000000006, 350.00000000000006, 352.0, 354.0, 356.0, 358.0, 360.0, 362.0, 364.0, 366.0, 368.0, 370.0, 372.0, 374.0, 376.0, 378.0, 380.0, 382.0, 384.0, 386.0, 388.0, 390.0, 392.0, 394.0, 396.0, 398.0, 400.0, 402.0, 404.0, 406.0, 408.00000000000006, 410.00000000000006, 412.00000000000006, 414.00000000000006, 416.00000000000006, 418.0, 420.0, 422.0, 424.0, 426.0, 428.0, 430.0, 432.0, 434.0, 436.0, 438.0, 440.0, 442.0, 444.0, 446.0, 448.0, 450.0, 452.0, 454.0, 456.0, 458.0, 460.0, 462.0, 464.0, 466.0, 468.0, 470.00000000000006, 472.00000000000006, 474.00000000000006, 476.00000000000006, 478.00000000000006, 480.0, 482.0, 484.0, 486.0, 488.0, 490.0, 492.0, 494.0, 496.0, 498.0, 500.0, 502.0, 504.0, 506.0, 508.0, 510.0, 512.0, 514.0, 516.0, 518.0, 520.0, 522.0, 524.0, 526.0, 528.0, 530.0, 532.0, 534.0, 536.0, 538.0, 540.0, 542.0, 544.0, 546.0, 548.0, 550.0, 552.0, 554.0, 556.0, 558.0, 560.0, 562.0, 564.0, 566.0000000000001, 568.0000000000001, 570.0000000000001, 572.0000000000001, 574.0000000000001, 576.0000000000001, 578.0, 580.0, 582.0, 584.0, 586.0, 588.0, 590.0, 592.0, 594.0, 596.0, 598.0, 600.0, 602.0, 604.0, 606.0, 608.0, 610.0, 612.0, 614.0, 616.0, 618.0, 620.0, 622.0, 624.0, 626.0, 628.0, 630.0, 632.0, 634.0, 636.0, 638.0, 640.0, 642.0, 644.0, 646.0, 648.0, 650.0, 652.0, 654.0, 656.0, 658.0, 660.0, 662.0, 664.0, 666.0, 668.0], [0.030022268841845445, 0.032725709111965706, 0.023820771778676475, -0.001435712775982867, -0.043332264805232834, -0.09463569871932043, -0.13985627458656902, -0.15764865706551223, -0.12685466773188292, -0.0352698124404327, 0.1122301694907808, 0.28885586554737763, 0.4465250665220184, 0.5264070093712565, 0.47009199991315853, 0.23052812921537402, -0.20822226661661603, -0.8201923549902261, -1.5401528046732746, -2.271848987778622, -2.9039839589873786, -3.330647410546968, -3.471897873769711, -3.290477950393882, -2.801120711558802, -2.070458731265168, -1.2073571897720043, -0.3453560034853851, 0.38233702029625505, 0.8603717960406705, 1.0106063479392695, 0.8122105959719264, 0.29662788405511975, -0.45768706605200293, -1.333071129950806, -2.1946969382524806, -2.908807318588451, -3.3648555943896383, -3.4971125676281396, -3.2903301364873982, -2.778533696410431, -2.045004426785585, -1.2130904472451451, -0.42087694739043435, 0.20720704275115587, 0.5783399668172589, 0.6467988251029038, 0.42594907629631784, -0.020570721543869297, -0.6002747311936751, -1.212323265979375, -1.7644348408877484, -2.191745186265333, -2.47509419745594, -2.6345560739984535, -2.709848052371102, -2.7514654828294365, -2.808551442233963, -2.915810436103307, -3.093597222859472, -3.344592491204276, -3.656877940857174, -4.019876948355124, -4.418416806089832, -4.834917473450025, -5.261303249126649, -5.691102519901458, -6.11847361410662, -6.54085106961352, -6.962416724867592, -7.3967587148317, -7.86151965021638, -8.379347813840837, -8.977671102746376, -9.681452317446578, -10.50795660731036, -11.460942465241981, -12.53080308059236, -13.691085903343575, -14.907942694256965, -16.15347176226468, -17.397161032407702, -18.623256009324287, -19.84877010671063, -21.112371818778264, -22.464425376182, -23.95959320525521, -25.648433118334594, -27.564763506122688, -29.715889495575784, -32.07904507899815, -34.604399101394364, -37.23071065015121, -39.904099731661525, -42.58456965099256, -45.25354570041664, -47.92306403108061, -50.634658439485214, -53.451366598273495, -56.43473266867364, -59.63127497187579, -63.05838635117463, -66.69179101630617, -70.47855526353698, -74.34237836002224, -78.19508035763604, -81.96886220089985, -85.63158756368301, -89.1874883153555, -92.6858343474089, -96.20855649018625, -99.84000877397159, -103.64869169933435, -107.66870373266842, -111.88926835740037, -116.25545060006617, -120.67502295928011, -125.03804327708767, -129.23665472749963, -133.18469690528877, -136.830366711188, -140.15566918805126, -143.18241990125318, -145.9685077937073, -148.5865497583277, -151.10899192034304, -153.59269573617868, -156.05913293568688, -158.47900771747265, -160.77529700766988, -162.83332839978274, -164.5131678072201, -165.68392603370208, -166.26079175898235, -166.22573239653798, -165.632557524701, -164.60564322152865, -163.3188618919035, -161.945869947698, -160.6204871391407, -159.41258150338234, -158.3008437735101, -157.17210567458935, -155.8600659164365, -154.17789052977992, -151.9525659396703, -149.06710426335053, -145.47873286837228, -141.22654603247537, -136.41660625349908, -131.1866127673058, -125.67576849634368, -120.00306704006162, -114.25108534771474, -108.45729810855117, -102.63241626190928, -96.78168262923698, -90.90497523843642, -85.00080146230778, -79.07831396825239, -73.15501513167058, -67.23880099839312, -61.32344570306634, -55.4045423761511, -49.484752232028654, -43.57701735616317, -37.7151976891989, -31.9567754573578, -26.37483192510303, -21.04725679398041, -16.044853968728997, -11.411941239539715, -7.158954523291953, -3.273134307580066, 0.27316885049611717, 3.516691606046016, 6.491402045283291, 9.220982525126026, 11.717665724953523, 13.981985798695238, 16.015054373562435, 17.823687101028206, 19.41465592679789, 20.797699615256256, 21.98223898366095, 22.976210786367293, 23.775873525243156, 24.36370455652305, 24.72715321382001, 24.862774789657397, 24.772951667892006, 24.476068413116202, 